vi "Controle_Manip_Main_GUI_WorkingBackup_211222.vi"() -> ()   [LabVIEW 2019] (continued)
            n2409 = event-data() -> ("CtlRef"=w2881:refnum<vi>, "NewVal"=w2879:dbl)  [unwired: 1 in, 4 out]
            n2410 = local read "Att Mode"() -> (w2880:enum16{"Single Step", "Continuous", "Automatic"})
            n2411 = flat-sequence {
              tunnel: w2881 -> [w2884]
              tunnel: w2880 -> [w2883]
              tunnel: w2879 -> [w2882]
              frame #0 {
                n2412 = case shown="\"Automatic\"" w2883 {
                  tunnel: w2884 -> [_ w2894]
                  tunnel: w2882 -> [_ w2892]
                  frame "Single Step", Default {
                  }
                  frame "Automatic" {
                    n2413 = property class="DigNum (strict)"(reference=w2894) -> ("Label.Text"=w2893:string)  [unwired: 1 in, 2 out]
                    n2414 = local read "Att DeviceHandle"() -> (w2888:u64)
                    n2415 = local read "Att Error"() -> (w2887:errorcluster)
                    n2416 = case shown="\"Att Pos X\", Default" w2893 {
                      tunnel: [w2896 w2898 w2900] -> w2891
                      tunnel: [w2895 w2897 w2899] -> _
                      frame "Att Pos X", Default {
                        w2896 = u8 1 items=["1", "2", "3"] ("axis")
                        n2417 = control-ref of="Att Pos X"() -> (w2895:refnum<vi>)
                      }
                      frame "Att Pos Y" {
                        w2898 = u8 0 items=["1", "2", "3"] ("axis")
                        n2418 = control-ref of="Att Pos Y"() -> (w2897:refnum<vi>)
                      }
                      frame "Att Pos Z" {
                        w2900 = u8 2 items=["1", "2", "3"] ("axis")
                        n2419 = control-ref of="Att Pos Z"() -> (w2899:refnum<vi>)
                      }
                    }
                    n2420 = local read "ourDLL"() -> (w2889:path)
                    n2421 = call "ANC_MoveAbs.vi"("Att DeviceHandle"=w2888, "ourDLL"=w2889, "axis"=w2891, "Target pos"=w2892, "Att Error"=w2887) -> ("deviceHandle out"=w2886:u64, "Out Position [µm | m°]"=→"Out Position [µm | m°]":dbl, "error out"=w2885:errorcluster)  [unwired: 1 in]
                    n2422 = local write "Att DeviceHandle"(w2886) -> ()
                    n2423 = local write "Att Error"(w2885) -> ()
                  }
                }
              }
              frame #1 {
                n2424 = property on="Att Read Pos" class="Bool (strict)"("Val(Sgnl)"=TRUE ("Value (Signaling)")) -> ()  [unwired: 2 in, 2 out]
              }
            }
          }
          event "Att Read Pos": Value Change {
            n2425 = event-data() -> ()  [unwired: 1 in, 6 out]
            n2426 = flat-sequence {
              frame #0 {
                w2902 = u8 2 items=["1", "2", "3"] ("axis")
                w2903 = u8 1 items=["1", "2", "3"] ("axis")
                w2904 = u8 0 items=["1", "2", "3"] ("axis")
                n2427 = local read "Att DeviceHandle"() -> (w2916:u64)
                n2428 = local read "Att Error"() -> (w2915:errorcluster)
                n2429 = local read "ourDLL"() -> (w2910:path)
                n2430 = call "ANC350v4_GetPosition.vi"("deviceHandle"=w2916, "Path to *.DLL"=w2910, "axis"=w2904, "error in"=w2915) -> ("deviceHandle"=w2914:u64, "Position [µm | m°]"=w2909:dbl, "error ANC350v4_getPosition"=w2913:errorcluster)  [unwired: 8 in, 1 out]
                n2431 = call "ANC350v4_GetPosition.vi"("deviceHandle"=w2914, "Path to *.DLL"=w2910, "axis"=w2903, "error in"=w2913) -> ("deviceHandle"=w2912:u64, "Position [µm | m°]"=w2908:dbl, "error ANC350v4_getPosition"=w2911:errorcluster)  [unwired: 8 in, 1 out]
                n2432 = local write "Att Pos Y"(w2909) -> ()
                n2433 = local write "Att Pos X"(w2908) -> ()
                n2434 = call "ANC350v4_GetPosition.vi"("deviceHandle"=w2912, "Path to *.DLL"=w2910, "axis"=w2902, "error in"=w2911) -> ("deviceHandle"=w2906:u64, "Position [µm | m°]"=w2907:dbl, "error ANC350v4_getPosition"=w2905:errorcluster)  [unwired: 8 in, 1 out]
                n2435 = local write "Att DeviceHandle"(w2906) -> ()
                n2436 = local write "Att Pos Z"(w2907) -> ()
                n2437 = local write "Att Error"(w2905) -> ()
              }
              frame #1 {
                n2438 = local write "Att Read Pos"(FALSE ("Att Read Pos")) -> ()
              }
            }
          }
          event "Att Track Target": Value Change {
            n2439 = event-data() -> ("NewVal"=w2918:bool)  [unwired: 1 in, 5 out]
            n2440 = case shown="False" w2918 {
              frame False {
                w2929 = u8 2 items=["1", "2", "3"] ("axis")
                w2930 = u8 1 items=["1", "2", "3"] ("axis")
                w2935 = u8 0 items=["1", "2", "3"] ("axis")
                n2441 = local read "Att DeviceHandle"() -> (w2923:u64)
                n2442 = local read "Att Error"() -> (w2922:errorcluster)
                n2443 = local read "ourDLL"() -> (w2919:path)
                n2444 = call "ANC350v4_StartAutoMove.vi"("deviceHandle"=w2923, "Path to *.DLL"=w2919, "axis"=w2935, "Enable | Disable"=FALSE, "Relative | Absolute"=TRUE, "error in"=w2922) -> ("deviceHandle out"=w2934:u64, "error ANC350v4_StartAutoMove"=w2933:errorcluster)  [unwired: 7 in, 1 out]
                n2445 = call "ANC350v4_StartAutoMove.vi"("deviceHandle"=w2934, "Path to *.DLL"=w2919, "axis"=w2930, "Enable | Disable"=FALSE, "Relative | Absolute"=TRUE, "error in"=w2933) -> ("deviceHandle out"=w2932:u64, "error ANC350v4_StartAutoMove"=w2931:errorcluster)  [unwired: 7 in, 1 out]
                n2446 = call "ANC350v4_StartAutoMove.vi"("deviceHandle"=w2932, "Path to *.DLL"=w2919, "axis"=w2929, "Enable | Disable"=FALSE, "Relative | Absolute"=TRUE, "error in"=w2931) -> ("deviceHandle out"=w2921:u64, "error ANC350v4_StartAutoMove"=w2920:errorcluster)  [unwired: 7 in, 1 out]
                n2447 = local write "Att DeviceHandle"(w2921) -> ()
                n2448 = local write "Att Error"(w2920) -> ()
              }
              frame True {
              }
            }
          }
          event "Att Up", "Att Down", "Att Left", "Att Right", "Att Backward", "Att Forward": Value Change {
            n2449 = event-data() -> ("CtlRef"=w2938:refnum<vi>, "NewVal"=w2939:bool)  [unwired: 1 in, 4 out]
            n2450 = local read "Voltage Output?"() -> (w2937:bool)
            n2451 = case shown="True" w2937 {
              tunnel: w2939 -> [_ w2942]
              tunnel: w2938 -> [_ w2941]
              frame False {
              }
              frame True {
                n2452 = local read "Att DeviceHandle"() -> (w2947:u64)
                n2453 = local read "ourDLL"() -> (w2944:path)
                n2454 = local read "Att Error"() -> (w2946:errorcluster)
                n2455 = local read "Att Mode"() -> (w2948:enum16{"Single Step", "Continuous", "Automatic"})
                n2456 = property class="Bool (strict)"(reference=w2941) -> ("Label.Text"=w2945:string)  [unwired: 1 in, 2 out]
                n2457 = case shown="\"Automatic\"" w2948 {
                  tunnel: w2947 -> [w2952 w2990 w3037]
                  tunnel: w2946 -> [w2953 w2991 w3036]
                  tunnel: w2945 -> [w2951 w2994 w3018]
                  tunnel: w2944 -> [w2957 w2987 w3029]
                  tunnel: [w2956 w2997 w3041] -> w2943
                  tunnel: [w2955 w2996 w3040] -> w2940
                  tunnel: w2942 -> [_ w2993 _]
                  tunnel: w2941 -> [_ _ w3021]
                  frame "Single Step", Default {
                    n2458 = case shown="\"Att Up\"" w2951 {
                      tunnel: [FALSE ("direction [t=bwd | f=fwd]") TRUE FALSE ("direction [t=bwd | f=fwd]") TRUE ("direction [t=bwd | f=fwd]") FALSE ("direction [t=bwd | f=fwd]") TRUE ("direction [t=bwd | f=fwd]")] -> w2960
                      tunnel: [w2973 w2975 w2978 w2979 w2982 w2983] -> w2954
                      frame "Att Forward" {
                        w2973 = u8 2 items=["1", "2", "3"] ("axis")
                      }
                      frame "Att Backward" {
                        w2975 = u8 2 items=["1", "2", "3"] ("axis")
                      }
                      frame "Att Up" {
                        w2978 = u8 0 items=["1", "2", "3"] ("axis")
                      }
                      frame "Att Down", Default {
                        w2979 = u8 0 items=["1", "2", "3"] ("axis")
                      }
                      frame "Att Left" {
                        w2982 = u8 1 items=["1", "2", "3"] ("axis")
                      }
                      frame "Att Right" {
                        w2983 = u8 1 items=["1", "2", "3"] ("axis")
                      }
                    }
                    n2459 = call "ANC350v4_SingleStep.vi"("deviceHandle"=w2952, "Path to *.DLL"=w2957, "axis"=w2954, "direction [t=bwd | f=fwd]"=w2960, "error in"=w2953) -> ("deviceHandle"=w2958:u64, "error ANC350v4_singleStep"=w2959:errorcluster)  [unwired: 8 in, 1 out]
                    n2460 = call "ANC350v4_GetPosition.vi"("deviceHandle"=w2958, "Path to *.DLL"=w2957, "axis"=w2954, "error in"=w2959) -> ("deviceHandle"=w2956:u64, "Position [µm | m°]"=w2950:dbl, "error ANC350v4_getPosition"=w2955:errorcluster)  [unwired: 8 in, 1 out]
                    n2461 = case shown="\"Att Backward\"" w2951 {
                      tunnel: w2950 -> [w2962 w2964 w2966 w2968 w2970 _ w2972]
                      tunnel: FALSE -> [w2961 w2963 w2965 w2967 w2969 _ w2971]
                      frame "Att Right" {
                        n2462 = local write "Att Right"(w2961) -> ()
                        n2463 = local write "Att Pos X"(w2962) -> ()
                      }
                      frame "Att Left" {
                        n2464 = local write "Att Left"(w2963) -> ()
                        n2465 = local write "Att Pos X"(w2964) -> ()
                      }
                      frame "Att Up" {
                        n2466 = local write "Att Up"(w2965) -> ()
                        n2467 = local write "Att Pos Y"(w2966) -> ()
                      }
                      frame "Att Down" {
                        n2468 = local write "Att Down"(w2967) -> ()
                        n2469 = local write "Att Pos Y"(w2968) -> ()
                      }
                      frame "Att Forward" {
                        n2470 = local write "Att Forward"(w2969) -> ()
                        n2471 = local write "Att Pos Z"(w2970) -> ()
                      }
                      frame "False", Default {
                      }
                      frame "Att Backward" {
                        n2472 = local write "Att Backward"(w2971) -> ()
                        n2473 = local write "Att Pos Z"(w2972) -> ()
                      }
                    }
                  }
                  frame "Continuous" {
                    n2474 = case shown="False" w2993 {
                      tunnel: [FALSE TRUE] -> w2988
                      frame False {
                      }
                      frame True {
                      }
                    }
                    n2475 = case shown="\"Att Left\"" w2994 {
                      tunnel: [FALSE ("direction [t=bwd | f=fwd]") TRUE FALSE ("direction [t=bwd | f=fwd]") TRUE ("direction [t=bwd | f=fwd]") FALSE ("direction [t=bwd | f=fwd]") TRUE ("direction [t=bwd | f=fwd]")] -> w2992
                      tunnel: [w3006 w3008 w3011 w3012 w3015 w3016] -> w2989
                      frame "Att Forward" {
                        w3006 = u8 2 items=["1", "2", "3"] ("axis")
                      }
                      frame "Att Backward" {
                        w3008 = u8 2 items=["1", "2", "3"] ("axis")
                      }
                      frame "Att Up" {
                        w3011 = u8 0 items=["1", "2", "3"] ("axis")
                      }
                      frame "Att Down", Default {
                        w3012 = u8 0 items=["1", "2", "3"] ("axis")
                      }
                      frame "Att Left" {
                        w3015 = u8 1 items=["1", "2", "3"] ("axis")
                      }
                      frame "Att Right" {
                        w3016 = u8 1 items=["1", "2", "3"] ("axis")
                      }
                    }
                    n2476 = call "ANC350v4_StartContinousMove.vi"("deviceHandle"=w2990, "Path to *.DLL"=w2987, "axis"=w2989, "start | stop"=w2988, "direction [t=bwd | f=fwd]"=w2992, "error in"=w2991) -> ("deviceHandle"=w2985:u64, "error ANC350v4_startContinousMove"=w2986:errorcluster)  [unwired: 7 in, 1 out]
                    n2477 = call "ANC350v4_GetPosition.vi"("deviceHandle"=w2985, "Path to *.DLL"=w2987, "axis"=w2989, "error in"=w2986) -> ("deviceHandle"=w2997:u64, "Position [µm | m°]"=w2995:dbl, "error ANC350v4_getPosition"=w2996:errorcluster)  [unwired: 8 in, 1 out]
                    n2478 = case shown="\"Att Right\"" w2994 {
                      tunnel: w2995 -> [_ w3000 w3001 w3002 w3003 w3004 w3005]
                      frame "False", Default {
                      }
                      frame "Att Right" {
                        n2479 = local write "Att Pos X"(w3000) -> ()
                      }
                      frame "Att Left" {
                        n2480 = local write "Att Pos X"(w3001) -> ()
                      }
                      frame "Att Up" {
                        n2481 = local write "Att Pos Y"(w3002) -> ()
                      }
                      frame "Att Down" {
                        n2482 = local write "Att Pos Y"(w3003) -> ()
                      }
                      frame "Att Forward" {
                        n2483 = local write "Att Pos Z"(w3004) -> ()
                      }
                      frame "Att Backward" {
                        n2484 = local write "Att Pos Z"(w3005) -> ()
                      }
                    }
                  }
                  frame "Automatic" {
                    n2485 = local read "Att AutoStep"() -> (w3019:dbl)
                    n2486 = case shown="\"Att Right\"" w3018 {
                      tunnel: [w3083 w3086 w3088 w3091 w3093 w3096] -> w3030
                      tunnel: [w3082 w3084 w3087 w3090 w3092 w3094] -> w3020
                      tunnel: w3019 -> [w3082 w3085 w3087 w3089 w3092 w3095]
                      frame "Att Forward" {
                        w3083 = u8 2 items=["1", "2", "3"] ("axis")
                      }
                      frame "Att Backward" {
                        w3086 = u8 2 items=["1", "2", "3"] ("axis")
                        n2487 = Negate(x=w3085) -> (-x=w3084:dbl)
                      }
                      frame "Att Up" {
                        w3088 = u8 0 items=["1", "2", "3"] ("axis")
                      }
                      frame "Att Down", Default {
                        w3091 = u8 0 items=["1", "2", "3"] ("axis")
                        n2488 = Negate(x=w3089) -> (-x=w3090:dbl)
                      }
                      frame "Att Left" {
                        w3093 = u8 1 items=["1", "2", "3"] ("axis")
                      }
                      frame "Att Right" {
                        w3096 = u8 1 items=["1", "2", "3"] ("axis")
                        n2489 = Negate(x=w3095) -> (-x=w3094:dbl)
                      }
                    }
                    n2490 = call "ANC350v4_SetTarget.vi"("deviceHandle"=w3037, "Path to *.DLL"=w3029, "axis"=w3030, "Target [µm | m°]"=w3020, "error in"=w3036) -> ("deviceHandle"=w3038:u64, "error ANC350v4_setTarget"=w3035:errorcluster)  [unwired: 8 in, 1 out]
                    n2491 = call "ANC350v4_StartAutoMove.vi"("deviceHandle"=w3038, "Path to *.DLL"=w3029, "axis"=w3030, "Enable | Disable"=TRUE, "Relative | Absolute"=TRUE, "error in"=w3035) -> ("deviceHandle out"=w3031:u64, "error ANC350v4_StartAutoMove"=w3032:errorcluster)  [unwired: 7 in, 1 out]
                    n2492 = while {
                      tunnel: w3032 -> [w3075]
                      tunnel: w3031 -> [w3074]
                      tunnel: w3030 -> [w3064]
                      tunnel: w3029 -> [w3063]
                      tunnel: [w3067] -> w3025
                      tunnel: [w3066] -> w3024
                      tunnel: [w3063] -> w3023
                      tunnel: [w3064] -> w3022
                      tunnel: w3018 -> [w3062]
                      stop <- w3071 stop-if-true
                      n2493 = call "ANC350v4_GetAxisStatus.vi"("deviceHandle"=w3074, "Path to *.DLL"=w3063, "axis"=w3064, "error in"=w3075) -> ("deviceHandle"=w3068:u64, "Target"=w3072:bool, "error ANC350v4_getAxisStatus"=w3065:errorcluster)  [unwired: 6 in, 3 out]
                      n2494 = Wait (ms)(milliseconds to wait=u32 250) -> ()  [unwired: 1 out]
                      n2495 = call "ANC350v4_GetPosition.vi"("deviceHandle"=w3068, "Path to *.DLL"=w3063, "axis"=w3064, "error in"=w3065) -> ("deviceHandle"=w3067:u64, "Position [µm | m°]"=w3069:dbl, "error ANC350v4_getPosition"=w3066:errorcluster)  [unwired: 8 in, 1 out]
                      n2496 = case shown="\"Att Down\"" w3062 {
                        tunnel: w3069 -> [_ w3076 w3077 w3078 w3079 w3080 w3081]
                        frame "False", Default {
                        }
                        frame "Att Right" {
                          n2497 = local write "Att Pos X"(w3076) -> ()
                        }
                        frame "Att Left" {
                          n2498 = local write "Att Pos X"(w3077) -> ()
                        }
                        frame "Att Up" {
                          n2499 = local write "Att Pos Y"(w3078) -> ()
                        }
                        frame "Att Down" {
                          n2500 = local write "Att Pos Y"(w3079) -> ()
                        }
                        frame "Att Forward" {
                          n2501 = local write "Att Pos Z"(w3080) -> ()
                        }
                        frame "Att Backward" {
                          n2502 = local write "Att Pos Z"(w3081) -> ()
                        }
                      }
                      n2503 = Or(x=w3072, y="Att Stop Target Wait") -> (x .or. y?=w3071:bool)
                    }
                    n2504 = local read "Att Track Target"() -> (w3026:bool)
                    n2505 = case shown="False" w3026 {
                      tunnel: w3025 -> [w3058 w3061]
                      tunnel: w3024 -> [w3057 w3060]
                      tunnel: [w3055 w3061] -> w3028
                      tunnel: [w3056 w3060] -> w3027
                      tunnel: w3023 -> [w3059 _]
                      tunnel: w3022 -> [w3054 _]
                      frame False {
                        n2506 = call "ANC350v4_StartAutoMove.vi"("deviceHandle"=w3058, "Path to *.DLL"=w3059, "axis"=w3054, "Enable | Disable"=FALSE, "Relative | Absolute"=TRUE, "error in"=w3057) -> ("deviceHandle out"=w3055:u64, "error ANC350v4_StartAutoMove"=w3056:errorcluster)  [unwired: 7 in, 1 out]
                      }
                      frame True {
                      }
                    }
                    n2507 = call "ANC350v4_GetPosition.vi"("deviceHandle"=w3028, "Path to *.DLL"=w3029, "axis"=w3030, "error in"=w3027) -> ("deviceHandle"=w3041:u64, "Position [µm | m°]"=w3039:dbl, "error ANC350v4_getPosition"=w3040:errorcluster)  [unwired: 8 in, 1 out]
                    n2508 = stacked-sequence {
                      tunnel: w3039 -> [w3043 _]
                      tunnel: w3018 -> [w3042 _]
                      tunnel: w3021 -> [_ w3050]
                      frame #0 {
                        n2509 = case shown="\"Att Right\"" w3042 {
                          tunnel: w3043 -> [_ w3044 w3045 w3046 w3047 w3048 w3049]
                          frame "False", Default {
                          }
                          frame "Att Right" {
                            n2510 = local write "Att Pos X"(w3044) -> ()
                          }
                          frame "Att Left" {
                            n2511 = local write "Att Pos X"(w3045) -> ()
                          }
                          frame "Att Up" {
                            n2512 = local write "Att Pos Y"(w3046) -> ()
                          }
                          frame "Att Down" {
                            n2513 = local write "Att Pos Y"(w3047) -> ()
                          }
                          frame "Att Forward" {
                            n2514 = local write "Att Pos Z"(w3048) -> ()
                          }
                          frame "Att Backward" {
                            n2515 = local write "Att Pos Z"(w3049) -> ()
                          }
                        }
                      }
                      frame #1 {
                        n2516 = property class="Bool (strict)"(reference=w3050, "Value"=FALSE) -> ()  [unwired: 1 in, 2 out]
                      }
                    }
                  }
                }
                n2517 = local write "Att DeviceHandle"(w2943) -> ()
                n2518 = local write "Att Error"(w2940) -> ()
              }
            }
          }
          event "Att Wobble Get Pos 1", "Att Wobble Get Pos 2", "Att Wobble": Mouse Down {
            n2519 = event-data() -> ("CtlRef"=w3098:refnum<vi>)  [unwired: 1 in, 7 out]
            n2520 = property class="Bool (strict)"(reference=w3098) -> ("Label.Text"=w3097:string)  [unwired: 1 in, 2 out]
            n2521 = case shown="\"Att Wobble\"" w3097 {
              frame "Att Wobble" {
                n2522 = stacked-sequence {
                  frame #0 {
                    n2523 = local read "Att DeviceHandle"() -> (w3105:u64)
                    n2524 = local read "Att Wobble Start"() -> (w3107:dbl)
                    n2525 = local read "Att Wobble End"() -> (w3106:dbl)
                    n2526 = control-ref of="Att Wobble Stop2"() -> (w3100:refnum<vi>)
                    n2527 = local read "Att Error"() -> (w3104:errorcluster)
                    n2528 = local read "ourDLL"() -> (w3103:path)
                    n2529 = control-ref of="Att Pos Z"() -> (w3099:refnum<vi>)
                    n2530 = call "Att_Wobble.vi"("Att Pos Z"=w3099, "Att Wobble End"=w3106, "Att Wobble Start"=w3107, "Att Error"=w3104, "ourDLL"=w3103, "Att Wobble Stop2 2"=w3100, "Att DeviceHandle"=w3105) -> ("Att Error out"=w3101:errorcluster, "Att DeviceHandle out"=w3102:u64)  [unwired: 1 in]
                    n2531 = local write "Att DeviceHandle"(w3102) -> ()
                    n2532 = local write "Att Error"(w3101) -> ()
                  }
                  frame #1 {
                    w3108 = FALSE ("Att Wobble")
                    n2533 = local write "Att Wobble Stop2"(w3108) -> ()
                    n2534 = local write "Att Wobble"(w3108) -> ()
                  }
                }
              }
              frame "False", Default {
              }
              frame "Att Wobble Get Pos 1" {
                n2535 = property on="Att Pos Z" class="DigNum (strict)"() -> ("Value"=w3109:dbl)  [unwired: 2 in, 2 out]
                n2536 = local write "Att Wobble Start"(w3109) -> ()
              }
              frame "Att Wobble Get Pos 2" {
                n2537 = property on="Att Pos Z" class="DigNum (strict)"() -> ("Value"=w3110:dbl)  [unwired: 2 in, 2 out]
                n2538 = local write "Att Wobble End"(w3110) -> ()
              }
            }
          }
          event "Auto< ?": Value Change {
            n2539 = event-data() -> ("NewVal"=w3111:bool)  [unwired: 1 in, 5 out]
            n2540 = case shown="True" w3111 {
              frame False {
                w3112 = TRUE ("Visible")
                n2541 = property on="Save Spectrum N" class="Bool (strict)"("Visible"=w3112) -> ()  [unwired: 2 in, 2 out]
                n2542 = property on="Save XY Map" class="Bool (strict)"("Visible"=w3112) -> ()  [unwired: 2 in, 2 out]
                n2543 = property on="Save Spectrum" class="Bool (strict)"("Visible"=w3112) -> ()  [unwired: 2 in, 2 out]
                n2544 = property on="Save PLE" class="Bool (strict)"("Visible"=w3112) -> ()  [unwired: 2 in, 2 out]
                n2545 = property on="Save fPow" class="Bool (strict)"("Visible"=w3112) -> ()  [unwired: 2 in, 2 out]
                n2546 = property on="Save Custom Diode Spectrum" class="Bool (strict)"("Visible"=w3112) -> ()  [unwired: 2 in, 2 out]
                n2547 = property on="Save Michelson" class="Bool (strict)"("Visible"=w3112) -> ()  [unwired: 2 in, 2 out]
                n2548 = property on="Save Polarisation" class="Bool (strict)"("Visible"=w3112) -> ()  [unwired: 2 in, 2 out]
                n2549 = property on="Save Contrast" class="Bool (strict)"("Visible"=w3112) -> ()  [unwired: 2 in, 2 out]
              }
              frame True {
                w3113 = FALSE ("Visible")
                n2550 = property on="Save Spectrum N" class="Bool (strict)"("Visible"=w3113) -> ()  [unwired: 2 in, 2 out]
                n2551 = property on="Save XY Map" class="Bool (strict)"("Visible"=w3113) -> ()  [unwired: 2 in, 2 out]
                n2552 = property on="Save Spectrum" class="Bool (strict)"("Visible"=w3113) -> ()  [unwired: 2 in, 2 out]
                n2553 = property on="Save PLE" class="Bool (strict)"("Visible"=w3113) -> ()  [unwired: 2 in, 2 out]
                n2554 = property on="Save fPow" class="Bool (strict)"("Visible"=w3113) -> ()  [unwired: 2 in, 2 out]
                n2555 = property on="Save Polarisation" class="Bool (strict)"("Visible"=w3113) -> ()  [unwired: 2 in, 2 out]
                n2556 = property on="Save Michelson" class="Bool (strict)"("Visible"=w3113) -> ()  [unwired: 2 in, 2 out]
                n2557 = property on="Save Contrast" class="Bool (strict)"("Visible"=w3113) -> ()  [unwired: 2 in, 2 out]
                n2558 = property on="Save Custom Diode Spectrum" class="Bool (strict)"("Visible"=w3113) -> ()  [unwired: 2 in, 2 out]
              }
            }
          }
          event "Background substract": Value Change {
            n2559 = event-data() -> ("NewVal"=w3114:enum16{"None", "Shutter"})  [unwired: 1 in, 5 out]
            n2560 = case shown="\"Shutter\"" w3114 {
              frame "None", Default {
              }
              frame "Shutter" {
                n2561 = stacked-sequence {
                  tunnel: [_ _ w3164] -> w3115
                  frame #0 {
                    n2562 = local read "Log file"() -> (w3149:string)
                    n2563 = property on="CCD 1D Spectrum Main" class="XYGraph (strict)"("YScale.Offset"=0.0 ("Y Scale.Offset and Multiplier:Offset")) -> ()  [unwired: 2 in, 2 out]
                    n2564 = call "Write2LogFile.vi"("Add to log file"="Acquiring background", "Log file before"=w3149, "Checkbox"=FALSE) -> ("Log file after"=w3148:string)
                    n2565 = local write "Log file"(w3148) -> ()
                  }
                  frame #1 {
                    # "make sure shutter is closed"
                    n2566 = local read "KCube Shutter On?"() -> (w3150:bool)
                    n2567 = control-ref of="Shutter Ctrls"() -> (w3154:refnum<vi>)
                    n2568 = property class="Ring (strict)"(reference=w3154) -> ("Value"=w3153:u16)  [unwired: 1 in, 2 out]
                    n2569 = control-ref of="KCube Shutter Device Reference"() -> (w3155:refnum<vi>)
                    n2570 = Equal?(x=w3153, y=u16 0) -> (x = y?=w3151:bool)
                    n2571 = case shown="False" w3151 {
                      tunnel: w3155 -> [w3158 _]
                      tunnel: w3154 -> [w3157 _]
                      tunnel: w3150 -> [w3156 _]
                      frame False {
                        n2572 = call "Shutter.vi"("KCube Shutter Device Reference 2"=w3158, "Shutter Ctrls 2"=w3157, "Shutter on?"=w3156) -> ()
                      }
                      frame True {
                      }
                    }
                  }
                  frame #2 {
                    # "acquire"
                    n2573 = local read "LightField Automation error out"() -> (w3162:errorcluster)
                    n2574 = local read "LightField Automation out"() -> (w3163:refnum<class "LightField Automation.lvclass">)
                    n2575 = local read "Accumulations"() -> (w3159:dbl)
                    n2576 = call "LFA_Capture.vi"("error in (no error)"=w3162, "Frames"=w3159, "LightField Automation in"=w3163) -> ("error out"=w3161:errorcluster, "Data"=w3164:T26, "LightField Automation out"=w3160:refnum<class "LightField Automation.lvclass">)  [unwired: 6 in]
                    n2577 = local write "LightField Automation error out"(w3161) -> ()
                    n2578 = local write "LightField Automation out"(w3160) -> ()
                  }
                }
                n2579 = local read "Acq Mode"() -> (w3116:T3)
                n2580 = case shown="\"Spectrum\", Default" w3116 {
                  selector: w3116 -> [w3117 w3135]
                  tunnel: w3115 -> [w3118 w3136]
                  frame "Spectrum", Default {
                    n2581 = stacked-sequence {
                      tunnel: w3118 -> [_ w3129 _ _]
                      tunnel: w3117 -> [_ w3127 _ _]
                      frame #0 {
                        n2582 = property on="CCD 2D Image Main" class="IntGraph (strict)"("Visible"=FALSE) -> ()  [unwired: 2 in, 2 out]
                        n2583 = property on="CCD 1D Spectrum Main" class="XYGraph (strict)"("Visible"=TRUE) -> ()  [unwired: 2 in, 2 out]
                      }
                      frame #1 {
                        n2584 = local read "CCD ROI"() -> (w3122:T20)
                        n2585 = local read "Wavelength calibration"() -> (w3126:dbl[])
                        n2586 = Divide(x=1239.842, y=w3126) -> (x/y=w3124:dbl[])
                        n2587 = call "PrepareData4Graph.vi"("Wavelength nm"=w3124, "DataLF"=w3129, "CCD ROI"=w3122, "AcqMode"=w3127, "Data type"=T30."Spectre") -> ("Spectrum"=w3128:cluster{"Array 2":dbl[], "Array":dbl[]}, "PLInt out"=w3121:dbl[])  [unwired: 2 in, 2 out]
                        n2588 = local write "CCD 1D Spectrum Main"(w3128) -> ()
                        n2589 = local write "BackgroundSpec"(w3121) -> ()
                      }
                      frame #2 {
                        n2590 = local read "BackgroundSpec"() -> (w3130:dbl[])
                        n2591 = call-poly <vilib>:"Mean.vi"("X"=w3130) -> ("mean"=w3132:dbl)  [unwired: 1 out]
                        n2592 = Negate(x=w3132) -> (-x=w3131:dbl)
                        n2593 = property on="CCD 1D Spectrum Main" class="XYGraph (strict)"("YScale.Offset"=w3131) -> ()  [unwired: 2 in, 2 out]
                      }
                      frame #3 {
                        n2594 = local write "Background taken?"(TRUE ("Background taken?")) -> ()
                        n2595 = property on="Background substract" class="Enum (strict)"("Value"=enum16{"None", "Shutter"}."None" ("Background substract")) -> ()  [unwired: 2 in, 2 out]
                      }
                    }
                  }
                  frame "Image" {
                    n2596 = stacked-sequence {
                      tunnel: w3136 -> [_ w3144]
                      tunnel: w3135 -> [_ w3142]
                      frame #0 {
                        n2597 = property on="CCD 1D Spectrum Main" class="XYGraph (strict)"("Visible"=FALSE) -> ()  [unwired: 2 in, 2 out]
                        n2598 = property on="CCD 2D Image Main" class="IntGraph (strict)"("Visible"=TRUE) -> ()  [unwired: 2 in, 2 out]
                      }
                      frame #1 {
                        n2599 = local read "Wavelength calibration"() -> (w3143:dbl[])
                        n2600 = local read "CCD ROI"() -> (w3139:T20)
                        n2601 = call "PrepareData4Graph.vi"("Wavelength nm"=w3143, "DataLF"=w3144, "CCD ROI"=w3139, "AcqMode"=w3142, "Data type"=T30."Spectre") -> ("Intensity Graph"=w3141:dbl[][])  [unwired: 2 in, 3 out]
                        n2602 = local write "CCD 2D Image Main"(w3141) -> ()
                      }
                    }
                  }
                }
              }
            }
          }
          event "CCD 1D Spectrum Main  Cursor2WL 1 Mono 1", "CCD 1D Spectrum Main  Cursor2WL 2 Mono 1", "CCD 1D Spectrum Main  Cursor2WL 1 Mono 2", "CCD 1D Spectrum Main  Cursor2WL 2 Mono 2": Mouse Down {
            n2603 = event-data() -> ("CtlRef"=w3166:refnum<vi>)  [unwired: 1 in, 7 out]
            n2604 = property class="Bool (strict)"(reference=w3166) -> ("Label.Text"=w3165:string)  [unwired: 1 in, 2 out]
            n2605 = case shown="Default" w3165 {
              frame "CCD 1D Spectrum Main  Cursor2WL 1 Mono 1" {
                n2606 = local read "CCD 1D Spectrum Main Cursor 1 nm"() -> (w3167:dbl)
                n2607 = property on="Center Wavelength (nm)" class="DigNum (strict)"("Val(Sgnl)"=w3167) -> ()  [unwired: 2 in, 2 out]
              }
              frame "CCD 1D Spectrum Main  Cursor2WL 1 Mono 2" {
                n2608 = local read "CCD 1D Spectrum Main Cursor 1 nm"() -> (w3168:dbl)
                n2609 = property on="Mono2 Wavelength (nm)" class="DigNum (strict)"("Val(Sgnl)"=w3168) -> ()  [unwired: 2 in, 2 out]
              }
              frame "CCD 1D Spectrum Main  Cursor2WL 2 Mono 2" {
                n2610 = local read "CCD 1D Spectrum Main Cursor 2 nm"() -> (w3169:dbl)
                n2611 = property on="Mono2 Wavelength (nm)" class="DigNum (strict)"("Val(Sgnl)"=w3169) -> ()  [unwired: 2 in, 2 out]
              }
              frame "CCD 1D Spectrum Main  Cursor2WL 2 Mono 1" {
                n2612 = local read "CCD 1D Spectrum Main Cursor 2 nm"() -> (w3170:dbl)
                n2613 = property on="Center Wavelength (nm)" class="DigNum (strict)"("Val(Sgnl)"=w3170) -> ()  [unwired: 2 in, 2 out]
              }
              frame Default {
              }
            }
          }
          event "CCD 1D Spectrum Main", "Contrast Oscillations", "Contrast 1D Spectrum": Cursor Release {
            n2614 = event-data() -> ("CtlRef"=w3174:refnum<vi>, "CursRef"=w3172:refnum<vi>)  [unwired: 1 in, 7 out]
            n2615 = property class="XYGraph (strict)"(reference=w3174) -> ("Label.Text"=w3173:string)  [unwired: 1 in, 2 out]
            n2616 = property class="Curs"(reference=w3172) -> ("Cursor Name"=w3171:string)  [unwired: 1 in, 2 out]
            n2617 = case shown="\"Contrast 1D Spectrum\"" w3173 {
              tunnel: w3171 -> [w3175 _ _ _]
              frame "Contrast Oscillations" {
                n2618 = case shown="\"ContPos\"" w3175 {
                  frame "False", Default {
                  }
                  frame "ContPos" {
                    n2619 = local read "Cursor controls"() -> (w3176:bool)
                    n2620 = case shown="True" w3176 {
                      frame False {
                      }
                      frame True {
                        n2621 = property on="Contrast Oscillations" class="XYGraph (strict)"("Active Cursor"=u32 2) -> ("Cursor.Cursor X"=w3177:dbl)  [unwired: 2 in, 2 out]
                        n2622 = Number To Decimal String(number=w3177) -> (decimal integer string=w3179:string)  [unwired: 1 in]
                        n2623 = property on="Contrast 1D Spectrum from Cursors" class="XYGraph (strict)"("Caption.Text"=w3179) -> ()  [unwired: 2 in, 2 out]
                      }
                    }
                  }
                  frame "ContInt1" {
                    n2624 = property on="Contrast Oscillations" class="XYGraph (strict)"("Active Cursor"=u32 0, "Active Cursor"=u32 1) -> ("Cursor.Cursor Y"=w3182:dbl, "Cursor.Cursor Y"=w3181:dbl)  [unwired: 2 in, 2 out]
                    n2625 = call "Contrast.vi"("Y2"=w3181, "Y1"=w3182) -> ("(max(Y1,Y2) - min(Y1,Y2)) / (Y1 + Y2)"=w3180:dbl)
                    n2626 = local write "Contrast"(w3180) -> ()
                  }
                  frame "ContInt2" {
                    n2627 = property on="Contrast Oscillations" class="XYGraph (strict)"("Active Cursor"=u32 0, "Active Cursor"=u32 1) -> ("Cursor.Cursor Y"=w3187:dbl, "Cursor.Cursor Y"=w3186:dbl)  [unwired: 2 in, 2 out]
                    n2628 = call "Contrast.vi"("Y2"=w3186, "Y1"=w3187) -> ("(max(Y1,Y2) - min(Y1,Y2)) / (Y1 + Y2)"=w3185:dbl)
                    n2629 = local write "Contrast"(w3185) -> ()
                  }
                }
              }
              frame "Contrast 1D Spectrum" {
                n2630 = case shown="True" "Cursor controls" {
                  frame False {
                  }
                  frame True {
                    n2631 = property on="Contrast 1D Spectrum" class="XYGraph (strict)"("Active Cursor"=u32 0, "Active Cursor"=u32 1) -> ("Cursor.Cursor X"=w3198:dbl, "Cursor.Cursor X"=w3197:dbl)  [unwired: 2 in, 2 out]
                    n2632 = local read "Wavelength calibration"() -> (w3203:dbl[])
                    n2633 = local read "Contrast Array Out"() -> (w3199:dbl[][])
                    n2634 = Divide(x=1239.842, y=w3203) -> (x/y=w3200:dbl[])
                    n2635 = call "Cursors4Contrast_v2.vi"("Cursor 2"=w3197, "Cursor 1"=w3198, "Spectres vs PZA"=w3199, "Energy"=w3200) -> ("Contrast of ROI vs PZC"=w3196:dbl[], "Spectra ROI"=w3193:dbl[][], "Energy ROI"=w3195:dbl[])
                    n2636 = Index Array(array=w3193, index (row)=0) -> (element=w3191:dbl[])  [unwired: 1 in]
                    n2637 = local read "PZA12 Positions"() -> (w3202:dbl[])
                    n2638 = Bundle("Energy ROI"=w3195, "Spectra ROI"=w3191) -> (w3194:cluster{"Energy ROI":dbl[], "Spectra ROI":dbl[]})  [unwired: 1 in]
                    n2639 = property on="Contrast 1D Spectrum from Cursors" class="XYGraph (strict)"("Value"=w3194) -> ()  [unwired: 2 in, 2 out]
                    n2640 = Bundle("PZA12 Positions"=w3202, "Contrast of ROI vs PZC"=w3196) -> (w3201:T38)  [unwired: 1 in]
                    n2641 = property on="Contrast Oscillations" class="XYGraph (strict)"("Value"=w3201) -> ()  [unwired: 2 in, 2 out]
                  }
                }
              }
              frame Default {
              }
              frame "CCD 1D Spectrum Main" {
                n2642 = stacked-sequence {
                  seq-local: [w3208 _] -> [_ w3216]
                  seq-local: [w3207 _] -> [_ w3215]
                  frame #0 {
                    n2643 = property on="CCD 1D Spectrum Main" class="XYGraph (strict)"("Active Cursor"=u32 0, "Active Cursor"=u32 1) -> ("Cursor.Cursor X"=w3208:dbl, "Cursor.Cursor X"=w3207:dbl)  [unwired: 2 in, 2 out]
                    n2644 = local write "CCD 1D Spectrum Main Cursor"(w3208) -> ()
                    n2645 = local write "CCD 1D Spectrum Main Cursor 2"(w3207) -> ()
                  }
                  frame #1 {
                    n2646 = call "Cursors2Freq.vi"("Cursor 1 eV"=w3216, "Cursor 2 eV"=w3215) -> ("Cursor dE"=w3214:dbl, "Cursor 1 nm"=w3213:dbl, "Cursor 2 nm"=w3212:dbl, "Cursor dnm"=w3211:dbl)
                    n2647 = local write "CCD 1D Spectrum Main deltaE"(w3214) -> ()
                    n2648 = local write "CCD 1D Spectrum Main Cursor 1 nm"(w3213) -> ()
                    n2649 = local write "CCD 1D Spectrum Main Cursor 2 nm"(w3212) -> ()
                    n2650 = Multiply(x=w3211, y=1e-09) -> (x*y=w3217:dbl)
                    n2651 = local write "CCD 1D Spectrum Main deltanm"(w3217) -> ()
                  }
                }
              }
            }
          }
          event "CCD 1D Spectrum Main", "Polarisation 1D Spectrum", "CCD 1D Spectrum XY Map": Scale Range Change {
            n2652 = event-data() -> ("CtlRef"=w3219:refnum<vi>, "ScaleRef"=w3222:refnum<vi>, "NewRange"=w3220:T39)  [unwired: 1 in, 5 out]
            n2653 = property class="GrphScl"(reference=w3222) -> ("NameLbl.Text"=w3221:string)  [unwired: 1 in, 2 out]
            n2654 = case shown="\"Energy (eV)\"" w3221 {
              tunnel: w3219 -> [w3227 _]
              tunnel: w3220 -> [w3225 _]
              frame "Energy (eV)" {
                w3226 = 1239.842
                n2655 = property class="XYGraph (strict)"(reference=w3227) -> ("Label.Text"=w3230:string)  [unwired: 1 in, 2 out]
                n2656 = Unbundle By Name(w3225) -> ("Minimum"=w3224:dbl, "Maximum"=w3223:dbl)
                n2657 = Divide(x=w3226, y=w3224) -> (x/y=w3228:dbl)
                n2658 = Divide(x=w3226, y=w3223) -> (x/y=w3229:dbl)
                n2659 = case shown="\"CCD 1D Spectrum Main\", Default" w3230 {
                  tunnel: w3228 -> [w3235 w3261 w3267]
                  tunnel: w3229 -> [w3236 w3260 w3268]
                  tunnel: w3224 -> [w3231 w3257 _]
                  tunnel: w3223 -> [w3232 w3256 _]
                  frame "CCD 1D Spectrum Main", Default {
                    n2660 = disable-structure shown="Disabled" {
                      disable-tunnel: w3232 -> [w3238 _]
                      disable-tunnel: w3231 -> [w3237 _]
                      frame Disabled {
                        n2661 = property on="CCD 1D Spectrum Main" class="XYGraph (strict)"("Active Cursor"=1 ("Cursor.Cursor Index")) -> ("Cursor.Cursor X"=w3241:dbl)  [unwired: 2 in, 2 out]
                        n2662 = property on="CCD 1D Spectrum Main" class="XYGraph (strict)"("Active Cursor"=0 ("Cursor.Cursor Index")) -> ("Cursor.Cursor X"=w3243:dbl)  [unwired: 2 in, 2 out]
                        n2663 = In Range and Coerce(upper limit=w3238, x=w3243, lower limit=w3237) -> (In Range?=w3244:bool)  [unwired: 1 out]
                        n2664 = In Range and Coerce(upper limit=w3238, x=w3241, lower limit=w3237) -> (In Range?=w3240:bool)  [unwired: 1 out]
                        n2665 = Not(x=w3244) -> (.not. x?=w3245:bool)
                        n2666 = Not(x=w3240) -> (.not. x?=w3239:bool)
                        n2667 = case shown="True" w3245 {
                          tunnel: w3237 -> [_ w3249]
                          frame False {
                          }
                          frame True {
                            n2668 = property on="CCD 1D Spectrum Main" class="XYGraph (strict)"("Active Cursor"=0 ("Cursor.Cursor Index"), "Cursor.Cursor X"=w3249) -> ()  [unwired: 2 in, 2 out]
                          }
                        }
                        n2669 = case shown="True" w3239 {
                          tunnel: w3238 -> [_ w3247]
                          frame False {
                          }
                          frame True {
                            n2670 = property on="CCD 1D Spectrum Main" class="XYGraph (strict)"("Active Cursor"=1 ("Cursor.Cursor Index"), "Cursor.Cursor X"=w3247) -> ()  [unwired: 2 in, 2 out]
                          }
                        }
                      }
                      frame Enabled {
                      }
                    }
                    n2671 = property on="CCD 1D Spectrum Main Energy Scale" class="XYGraph (strict)"("XScale.Maximum"=w3235, "XScale.Minimum"=w3236, "XScale.UniformMarker"=TRUE ("X Scale.Uniform Marker Spacing?")) -> ()  [unwired: 2 in, 2 out]
                    n2672 = for {
                      N: 2 -> [_]
                      tunnel: w3232 -> [w3255]
                      tunnel: w3231 -> [w3254]
                      i -> [w3251]
                      # "coerce both cursors to new range"
                      n2673 = property on="CCD 1D Spectrum Main" class="XYGraph (strict)"("Active Cursor"=w3251) -> ("Cursor.Cursor X"=w3253:dbl)  [unwired: 2 in, 2 out]
                      n2674 = In Range and Coerce(upper limit=w3255, x=w3253, lower limit=w3254) -> (coerced(x)=w3252:dbl)  [unwired: 1 out]
                      n2675 = property on="CCD 1D Spectrum Main" class="XYGraph (strict)"("Active Cursor"=w3251, "Cursor.Cursor X"=w3252) -> ()  [unwired: 2 in, 2 out]
                    }
                  }
                  frame "CCD 1D Spectrum XY Map" {
                    n2676 = for {
                      N: 2 -> [_]
                      tunnel: w3257 -> [w3266]
                      tunnel: w3256 -> [w3265]
                      i -> [w3262]
                      # "coerce both cursors to new range"
                      n2677 = property on="CCD 1D Spectrum XY Map" class="XYGraph (strict)"("Active Cursor"=w3262) -> ("Cursor.Cursor X"=w3264:dbl)  [unwired: 2 in, 2 out]
                      n2678 = In Range and Coerce(upper limit=w3265, x=w3264, lower limit=w3266) -> (coerced(x)=w3263:dbl)  [unwired: 1 out]
                      n2679 = property on="CCD 1D Spectrum XY Map" class="XYGraph (strict)"("Active Cursor"=w3262, "Cursor.Cursor X"=w3263) -> ()  [unwired: 2 in, 2 out]
                    }
                    n2680 = property on="CCD 1D XY Map Spectrum Main Energy Scale" class="XYGraph (strict)"("XScale.Minimum"=w3260, "XScale.Maximum"=w3261, "XScale.UniformMarker"=TRUE ("X Scale.Uniform Marker Spacing?")) -> ()  [unwired: 2 in, 2 out]
                  }
                  frame "Polarisation 1D Spectrum" {
                    n2681 = property on="Polarisation 1D Spectrum Energy Scale" class="XYGraph (strict)"("XScale.Maximum"=w3267, "XScale.Minimum"=w3268) -> ()  [unwired: 2 in, 2 out]
                    n2682 = property on="CCD 1D XY Map Spectrum Main Energy Scale" class="XYGraph (strict)"("XScale.Minimum"=w3268, "XScale.Maximum"=w3267) -> ()  [unwired: 2 in, 2 out]
                  }
                }
              }
              frame "PL Intensity (cts)", Default {
              }
            }
          }
          event "Center Wavelength (nm)", "Mono2 Motor Pos", "Mono2 Wavelength (nm)": Value Change {
            n2683 = event-data() -> ("CtlRef"=w3270:refnum<vi>, "NewVal"=w3271:dbl)  [unwired: 1 in, 4 out]
            n2684 = property class="DigNum (strict)"(reference=w3270) -> ("Label.Text"=w3269:string)  [unwired: 1 in, 2 out]
            n2685 = case shown="\"Center Wavelength (nm)\", Default" w3269 {
              tunnel: w3271 -> [w3272 w3320 w3370]
              frame "Mono2 Motor Pos" {
                n2686 = local read "ESP 300 On?"() -> (w3273:bool)
                n2687 = case shown="True" w3273 {
                  tunnel: w3272 -> [_ w3276]
                  frame False {
                  }
                  frame True {
                    n2688 = control-ref of="Mono2 Motor Pos"() -> (w3275:refnum<vi>)
                    n2689 = control-ref of="Mono2 Wavelength (nm)"() -> (w3274:refnum<vi>)
                    n2690 = stacked-sequence {
                      tunnel: w3276 -> [_ w3284 _]
                      tunnel: w3275 -> [w3277 w3282 w3316]
                      tunnel: w3274 -> [w3278 w3281 w3317]
                      frame #0 {
                        # "disable controls when moving"
                        n2691 = property class="DigNum (strict)"(reference=w3278, "DisabledEnum"=T29."Disabled and Grayed Out" ("Disabled")) -> ()  [unwired: 1 in, 2 out]
                        n2692 = property class="DigNum (strict)"(reference=w3277, "DisabledEnum"=T29."Disabled and Grayed Out" ("Disabled")) -> ()  [unwired: 1 in, 2 out]
                      }
                      frame #1 {
                        # "move"
                        n2693 = local read "ESP300 COM Port"() -> (w3283:refnum<visa-resource-name>)
                        n2694 = disable-structure shown="Enabled" {
                          disable-tunnel: w3284 -> [w3292 w3308]
                          disable-tunnel: w3283 -> [w3288 w3309]
                          disable-tunnel: w3282 -> [w3285 w3310]
                          disable-tunnel: w3281 -> [_ w3306]
                          frame Disabled {
                            w3289 = 1 ("Axis")
                            n2695 = call "QMotor On.vi"("Axis"=w3289, "VISA resource name in"=w3288) -> ("error out"=w3295:errorcluster, "Motor On?"=w3297:bool, "VISA resource name out"=w3296:refnum<visa-resource-name>)  [unwired: 7 in]
                            n2696 = case shown="False" w3297 {
                              tunnel: w3289 -> [w3302 _]
                              tunnel: w3296 -> [w3301 w3304]
                              tunnel: w3295 -> [w3300 w3303]
                              tunnel: [w3299 w3304] -> w3294
                              tunnel: [w3298 w3303] -> w3293
                              frame False {
                                n2697 = call "Motor On.vi"("error in (no error)"=w3300, "Axis"=w3302, "VISA resource name in"=w3301) -> ("error out"=w3298:errorcluster, "VISA resource name out"=w3299:refnum<visa-resource-name>)  [unwired: 7 in]
                              }
                              frame True {
                              }
                            }
                            n2698 = call "Move To Position.vi"("error in (no error)"=w3293, "Postion (Unit)"=w3292, "Axis"=w3289, "VISA resource name in"=w3294) -> ("error out"=w3290:errorcluster, "VISA resource name out"=w3291:refnum<visa-resource-name>)  [unwired: 6 in]
                            n2699 = call "Wait For Motion Done.vi"("error in (no error)"=w3290, "Mono2 Motor Pos"=w3285, "Axis"=w3289, "VISA resource name"=w3291) -> ("error out"=w3286:errorcluster, "VISA resource name out"=w3287:refnum<visa-resource-name>)  [unwired: 6 in]
                            n2700 = local write "ESP300 COM Port"(w3287) -> ()
                            n2701 = local write "ESP300 Error"(w3286) -> ()
                          }
                          frame Enabled {
                            n2702 = local read "HR mode"() -> (w3305:u16)
                            n2703 = case shown="0, Default" w3305 {
                              tunnel: w3310 -> [w3315]
                              tunnel: w3309 -> [w3314]
                              tunnel: w3308 -> [w3313]
                              tunnel: w3306 -> [w3312]
                              tunnel: w3305 -> [w3311]
                              frame 0, Default {
                                n2704 = call "subVI_Mono2Go2Posv2.vi"("Mono2 Motor Pos"=w3315, "Mono2 Wavelength (nm)"=w3312, "HR mode"=w3311, "Postion (Unit)"=w3313, "ESP300 COM Port"=w3314) -> ()  [unwired: 2 out]
                              }
                            }
                            n2705 = call "MotorPos2WL.vi"("Mono2 Motor Position"=w3308, "HR mode"=w3305) -> ("Mono2 Center Wavelength (nm)"=w3307:dbl)
                            n2706 = local write "Mono2 Wavelength (nm)"(w3307) -> ()
                          }
                        }
                      }
                      frame #2 {
                        # "re-enable controls when finished moving"
                        n2707 = property class="DigNum (strict)"(reference=w3317, "DisabledEnum"=T29."Enabled" ("Disabled")) -> ()  [unwired: 1 in, 2 out]
                        n2708 = property class="DigNum (strict)"(reference=w3316, "DisabledEnum"=T29."Enabled" ("Disabled")) -> ()  [unwired: 1 in, 2 out]
                      }
                    }
                  }
                }
              }
              frame "Mono2 Wavelength (nm)" {
                n2709 = local read "ESP 300 On?"() -> (w3321:bool)
                n2710 = case shown="True" w3321 {
                  tunnel: w3320 -> [_ w3324]
                  frame False {
                  }
                  frame True {
                    n2711 = control-ref of="Mono2 Motor Pos"() -> (w3323:refnum<vi>)
                    n2712 = control-ref of="Mono2 Wavelength (nm)"() -> (w3322:refnum<vi>)
                    n2713 = stacked-sequence {
                      tunnel: w3324 -> [_ w3332 _]
                      tunnel: w3323 -> [w3328 w3331 w3367]
                      tunnel: w3322 -> [w3325 w3330 w3365]
                      frame #0 {
                        n2714 = property class="DigNum (strict)"(reference=w3328, "DisabledEnum"=T29."Disabled and Grayed Out" ("Disabled")) -> ()  [unwired: 1 in, 2 out]
                        n2715 = property class="DigNum (strict)"(reference=w3325, "DisabledEnum"=T29."Disabled and Grayed Out" ("Disabled")) -> ()  [unwired: 1 in, 2 out]
                      }
                      frame #1 {
                        n2716 = local read "HR mode"() -> (w3329:u16)
                        n2717 = local read "ESP300 COM Port"() -> (w3333:refnum<visa-resource-name>)
                        n2718 = disable-structure shown="Enabled" {
                          disable-tunnel: w3333 -> [w3337 w3358]
                          disable-tunnel: w3331 -> [w3334 w3359]
                          disable-tunnel: w3332 -> [_ w3357]
                          disable-tunnel: w3330 -> [_ w3355]
                          disable-tunnel: w3329 -> [_ w3354]
                          frame Disabled {
                            w3338 = 1 ("Axis")
                            n2719 = call "QMotor On.vi"("Axis"=w3338, "VISA resource name in"=w3337) -> ("error out"=w3344:errorcluster, "Motor On?"=w3346:bool, "VISA resource name out"=w3345:refnum<visa-resource-name>)  [unwired: 7 in]
                            n2720 = case shown="False" w3346 {
                              tunnel: w3338 -> [w3351 _]
                              tunnel: w3345 -> [w3350 w3353]
                              tunnel: w3344 -> [w3349 w3352]
                              tunnel: [w3348 w3353] -> w3343
                              tunnel: [w3347 w3352] -> w3342
                              frame False {
                                n2721 = call "Motor On.vi"("error in (no error)"=w3349, "Axis"=w3351, "VISA resource name in"=w3350) -> ("error out"=w3347:errorcluster, "VISA resource name out"=w3348:refnum<visa-resource-name>)  [unwired: 7 in]
                              }
                              frame True {
                              }
                            }
                            n2722 = call "Move To Position.vi"("error in (no error)"=w3342, "Axis"=w3338, "VISA resource name in"=w3343) -> ("error out"=w3339:errorcluster, "VISA resource name out"=w3340:refnum<visa-resource-name>, "Postion (Unit)"=w3341:dbl)  [unwired: 6 in]
                            n2723 = call "Wait For Motion Done.vi"("error in (no error)"=w3339, "Mono2 Motor Pos"=w3334, "Axis"=w3338, "VISA resource name"=w3340) -> ("error out"=w3335:errorcluster, "VISA resource name out"=w3336:refnum<visa-resource-name>)  [unwired: 6 in]
                            n2724 = local write "ESP300 COM Port"(w3336) -> ()
                            n2725 = local write "ESP300 Error"(w3335) -> ()
                          }
                          frame Enabled {
                            n2726 = call "MotorWL2Pos.vi"("Mono2 Center WL"=w3357, "HR mode"=w3354) -> ("Mono2 Position"=w3356:dbl)
                            n2727 = case shown="0, Default" w3354 {
                              tunnel: w3359 -> [w3364]
                              tunnel: w3358 -> [w3363]
                              tunnel: w3356 -> [w3362]
                              tunnel: w3355 -> [w3361]
                              tunnel: w3354 -> [w3360]
                              frame 0, Default {
                                n2728 = call "subVI_Mono2Go2Posv2.vi"("Mono2 Motor Pos"=w3364, "Mono2 Wavelength (nm)"=w3361, "HR mode"=w3360, "Postion (Unit)"=w3362, "ESP300 COM Port"=w3363) -> ()  [unwired: 2 out]
                              }
                            }
                            n2729 = local write "Mono2 Motor Pos"(w3356) -> ()
                          }
                        }
                      }
                      frame #2 {
                        n2730 = property class="DigNum (strict)"(reference=w3365, "DisabledEnum"=T29."Enabled" ("Disabled")) -> ()  [unwired: 1 in, 2 out]
                        n2731 = property class="DigNum (strict)"(reference=w3367, "DisabledEnum"=T29."Enabled" ("Disabled")) -> ()  [unwired: 1 in, 2 out]
                      }
                    }
                  }
                }
              }
              frame "Center Wavelength (nm)", Default {
                n2732 = local read "LightField On?"() -> (w3369:bool)
                n2733 = case shown="True" w3369 {
                  tunnel: w3370 -> [_ w3371]
                  frame False {
                  }
                  frame True {
                    n2734 = local read "LightField Automation error out"() -> (w3376:errorcluster)
                    n2735 = local read "LightField Automation out"() -> (w3377:refnum<class "LightField Automation.lvclass">)
                    n2736 = call "spec_GetCenterWavelength.vi"("error in (no error)"=w3376, "LightField Automation in"=w3377) -> ("error out"=w3372:errorcluster, "Center Wavelength"=w3375:dbl, "LightField Automation out"=w3373:refnum<class "LightField Automation.lvclass">)  [unwired: 7 in]
                    n2737 = Equal?(x=w3371, y=w3375) -> (x = y?=w3374:bool)
                    n2738 = case shown="False" w3374 {
                      tunnel: w3373 -> [w3380 w3392]
                      tunnel: w3372 -> [w3379 w3391]
                      tunnel: w3371 -> [w3378 _]
                      frame False {
                        n2739 = stacked-sequence {
                          tunnel: w3380 -> [_ w3384 _]
                          tunnel: w3379 -> [_ w3383 _]
                          tunnel: w3378 -> [_ w3382 _]
                          frame #0 {
                            w3381 = T29."Disabled and Grayed Out" ("Disabled")
                            n2740 = property on="Center Wavelength (nm)" class="DigNum (strict)"("DisabledEnum"=w3381) -> ()  [unwired: 2 in, 2 out]
                            n2741 = property on="Grating" class="CmbBox"("DisabledEnum"=w3381) -> ()  [unwired: 2 in, 2 out]
                            n2742 = property on="Exit mirror" class="Ring (strict)"("DisabledEnum"=w3381) -> ()  [unwired: 2 in, 2 out]
                          }
                          frame #1 {
                            n2743 = call "spec_SetCenterWavelength.vi"("error in (no error)"=w3383, "Center Wavelength"=w3382, "LightField Automation in"=w3384) -> ("error out"=w3388:errorcluster, "LightField Automation out"=w3389:refnum<class "LightField Automation.lvclass">)  [unwired: 7 in]
                            n2744 = call "spec_getCalibration.vi"("error in (no error)"=w3388, "LightField Automation in"=w3389) -> ("error out"=w3386:errorcluster, "ColumnCalibration"=w3387:dbl[], "LightField Automation out"=w3385:refnum<class "LightField Automation.lvclass">)  [unwired: 7 in]
                            n2745 = local write "LightField Automation error out"(w3386) -> ()
                            n2746 = local write "LightField Automation out"(w3385) -> ()
                            n2747 = local write "Wavelength calibration"(w3387) -> ()
                          }